vi "AeroQuadConfigurator.vi"() -> ()   [LabVIEW 2010]
uses:
  <vilib>/Utility/config.llb/Config Data RefNum.ctl
  <vilib>/Utility/miscctls.llb/LVRowAndColumnTypeDef.ctl
  <vilib>/Utility/miscctls.llb/LVRowAndColumnUnsignedTypeDef.ctl
  <vilib>/Utility/config.llb/Read Key (Double).vi
  <vilib>/Utility/config.llb/Read Key (String).vi
  <vilib>/Utility/config.llb/Read Key (I32).vi
  <vilib>/Utility/config.llb/Write Key (I32).vi
  <vilib>/Utility/config.llb/Write Key (String).vi
  <vilib>/Platform/browser.llb/Open URL in Default Browser (string).vi
  <vilib>/Instr/_visa.llb/VISA Configure Serial Port (Instr).vi
  <vilib>/Utility/config.llb/NI_LVConfig.lvlib
panel:
  out "LargeStatus":string
  in  "Load SubPanel":i32(ring) caption="Information Display" items=["Initial Setup", "3-D View", "Vehicle Status", "Mission Planner", "Motor Commands", "Serial Monitor", "Vehicle Attitude", "Sensor Data", "Transmitter Data"]
  in  "Parameter Type":i32(ring) caption="Configuration" items=["Rate Mode", "Attitude Mode", "Yaw Configuration", "Altitude Hold", "GPS Position Hold", "Miscellaneous Configuration", "Transmitter Smoothing", "Battery Monitor", "Camera Stabilization"]
  in  "Parameter Check":string[][](table)
  in  "Upload":bool
  out "Sensors":string[][](table)
  out "Status":string="AeroQuad Configurator"
  in  "*Com Port":refnum<visa-resource-name> caption="Com Port"
  in  "*Baud Rate":string(combo)="115200" caption="Baud Rate"
  in  "*BootDelay":dbl=3.0 caption="Boot Delay (s)"
  in  "*Timeout (sec)":dbl=3.0 caption="Timeout (s)"
  in  "Open Port":bool
  in  "Disconnect":bool
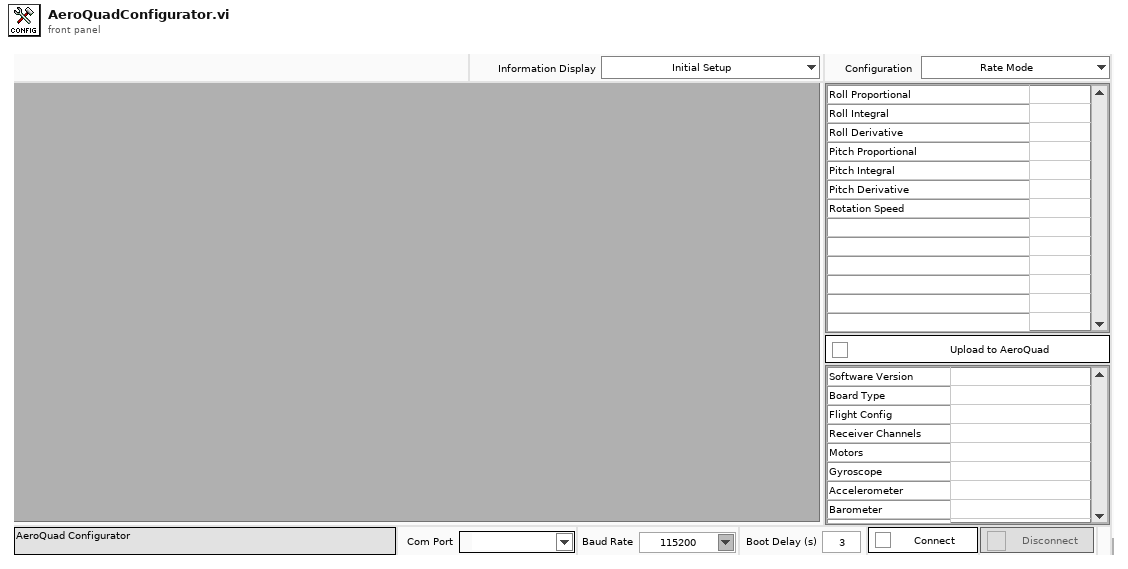
[diagram p1: front panel]
types:
  T1 = typedef "NI_LVConfig.lvlib/Config Data RefNum.ctl" = refnum<k1>
  T2 = cluster{"Error":errorcluster, "Data":dbl[], "COM Port":refnum<visa-resource-name>, "Data Type":enum16{"Serial", "Binary"}, "Connected":bool, "Parameters":string[][][], "WorkingPath":path, "ConfigRef":T1, "SubPanelName":string[], "ParameterName":string[], "Plots":string[][][], "SubPanelQueue":refnum<queue>, "SubPanel":refnum<vi>, "Debug":bool, "SubPanelType":string[], "Version":string, "StopTelem":string, "Config":string[][], "oldTelem":string, "previousValid":string, "oldCmd":string, "StartDelay":dbl, "ParamDesc":string[][], "IniPath":path, "SW":string, "ConnType":string, "ModemQueue":refnum<queue>, "Stale":i32, "Compatibility":dbl, "Logger":bool, "DebugLogger":refnum<queue>}
  T3 = enum8{"Enabled", "Disabled", "Disabled and Grayed Out"}
  T4 = cluster{"Section":string, "Key":string, "Value":string}
  T5 = enum32{"Invalid", "Standard", "Closed", "Hidden", "Minimized", "Maximized"}
  T6 = typedef "LVRowAndColumnTypeDef.ctl" = cluster{"Row":i32, "Column":i32}
  T7 = typedef "LVRowAndColumnUnsignedTypeDef.ctl" = cluster{"Row":u32, "Column":u32}
  T8 = enum32{"invalid app kind", "Development System", "Run Time System", "Student Edition", "Embedded LabVIEW", "Evaluation", "Custom"}
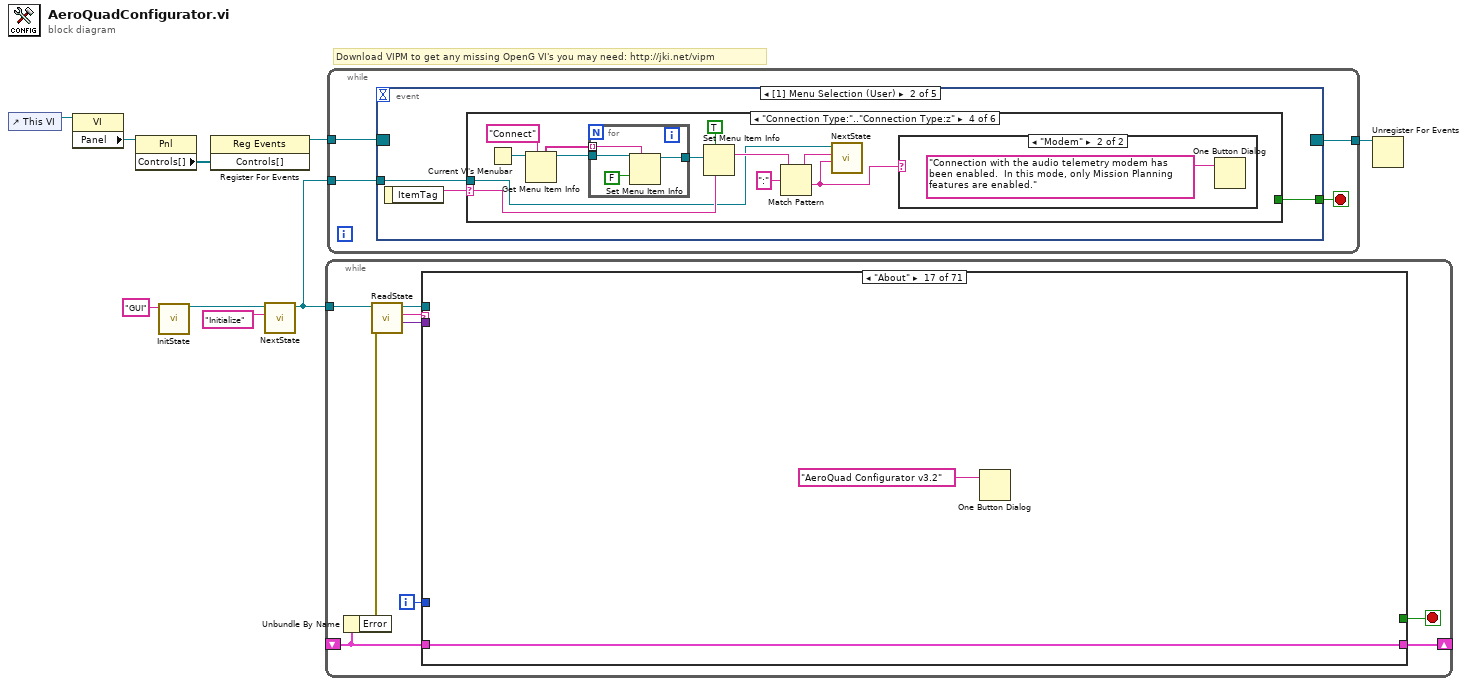
[diagram p0: block diagram]
diagram:
  # "Download VIPM to get any missing OpenG VI's you may need: http://jki.net/vipm"
  n1 = control-ref of="This VI"() -> (w9:refnum<vi>)
  n2 = property class="VI"(reference=w9) -> ("Panel"=w8:refnum<vi>)  [unwired: 1 in, 2 out]
  n3 = property class="Pnl"(reference=w8) -> ("Controls[]"=w7:refnum<vi>[])  [unwired: 1 in, 2 out]
  n4 = call "InitState.vi"("Name"="GUI") -> ("Queue Out"=w2:refnum<queue>)  [unwired: 8 in, 1 out]
  n5 = register-events(w7) -> (reference out=w6:refnum<event-registration>)  [unwired: 2 in, 1 out]
  n6 = call "NextState.vi"("State"="Initialize", "Queue In"=w2) -> ("Queue Out"=w3:refnum<queue>)  [unwired: 8 in, 1 out]
  n7 = while {
    tunnel: w3 -> [w13]
    shift-right: [w18] -> _
    shift-left: _ -> [w15]
    i -> [w16]
    stop <- w17 stop-if-true
    n8 = Unbundle By Name(w15) -> ("Error"=w14:errorcluster)
    n9 = call "ReadState.vi"("Error In"=w14, "Queue In"=w13) -> ("Data"=w10:variant, "State"=w11:string, "Queue Out"=w12:refnum<queue>)  [unwired: 6 in, 1 out]
    n10 = case shown="\"About\"" w11 {
      tunnel: w10 -> [_ _ _ w51 _ _ _ _ _ _ _ _ _ w251 w266 _ _ _ w323 w329 _ _ _ _ _ _ _ _ _ w492 w496 _ _ _ w667 _ _ _ w775 _ w785 _ _ w871 _ _ _ _ _ w1079 _ w1165 _ _ _ _ _ _ _ _ w1351 _ _ _ w1494 w1509 _ _ w1626 w1654 w1722]
      selector: w11 -> [_ w22 _ _ _ _ _ _ _ _ _ _ _ _ w256 _ _ _ _ _ _ _ _ _ _ _ _ _ _ _ _ _ _ _ w663 _ _ _ _ _ _ _ _ _ _ _ _ _ _ w1078 _ _ _ _ _ _ _ _ _ _ _ _ _ _ _ _ _ _ w1625 w1653 _]
      tunnel: [w19 w23 w36 w52 w56 w75 w111 w171 w187 w191 w193 w204 w240 w253 w267 w285 w317 w320 w324 w330 w332 w343 w346 w381 w436 w437 w470 w485 w487 w491 w497 w516 w544 w622 w668 w691 w726 w757 w772 w781 w787 w806 w818 w868 w903 w917 w949 w968 w1055 w1092 w1150 w1163 w1178 w1179 w1185 w1213 w1237 w1262 w1289 w1318 w1353 w1421 w1427 w1429 w1497 w1557 w1563 w1600 w1623 w1651 w1728] -> w18
      tunnel: [_ _ _ _ _ _ _ _ _ _ _ _ _ _ _ _ _ _ _ _ _ TRUE _ _ _ _ _ _ _ _ _ _ _ _ _ _ _ _ _ _ _ _ _ _ _ _ _ _ _ _ _ _ _ _ _ _ _ _ _ _ _ _ _ _ _ _ _ _ _ _ _] -> w17
      tunnel: w15 -> [w19 w23 _ w52 w56 w75 w112 w172 w188 w191 w193 w205 w241 w254 w267 w286 w317 w320 w324 w330 w332 w343 w346 w382 w436 w438 w470 w485 w487 w491 w497 w503 w545 w596 w669 w692 w727 w758 w772 w781 w788 w807 w819 w865 w903 w917 w949 w969 w1056 w1093 w1150 w1163 w1178 w1179 w1186 w1214 w1238 w1263 w1290 w1319 w1354 w1421 w1427 w1430 w1497 w1557 w1563 w1600 w1624 w1651 w1728]
      tunnel: w16 -> [_ _ _ _ _ _ _ _ _ _ _ _ _ _ _ w287 _ _ _ _ _ _ _ _ _ _ _ _ _ _ _ _ _ _ _ _ _ _ _ _ _ _ _ _ _ _ _ _ _ _ _ _ _ _ _ _ _ _ _ _ _ _ _ _ _ _ _ _ _ _ _]
      tunnel: w12 -> [_ _ w47 _ _ _ _ _ _ _ _ w198 w231 _ w260 w283 _ w319 _ _ _ w344 _ w355 _ _ _ _ _ _ w493 w508 w546 w621 w664 _ w725 w754 _ _ w789 w815 w825 w866 _ _ _ _ _ w1074 w1107 _ w1167 _ w1183 w1211 _ _ w1284 w1315 w1348 w1415 _ w1431 w1492 w1522 _ _ _ w1648 w1727]
      frame "--- System ---" {
      }
      frame Default {
        n11 = Format Into String(format string="Invalid state:\n%s", w22) -> (resulting string=w20:string)  [unwired: 2 in, 1 out]
        n12 = One Button Dialog(message=w20) -> ()  [unwired: 1 in, 1 out]
      }
      frame "Initialize" {
        w27 = "Launch" ("name (unnamed)")
        w28 = T3."Enabled" ("Disabled")
        # "Used for splash screen"
        n13 = call "NextState.vi"("Data"="Initializing Configurator", "State"="Status", "Queue In"=w47) -> ("Queue Out"=w30:refnum<queue>)  [unwired: 7 in, 1 out]
        n14 = call "NextStates.vi"("States"=string[] ["Lock Controls", "Load Config", "Load Parameters", "Load SubPanels", "Load Front Panel"], "Queue In"=w30) -> ("Queue Out"=w29:refnum<queue>)  [unwired: 8 in, 1 out]
        n15 = Current VI's Path() -> (path=w39:path)
        n16 = property class="App"() -> ("App.Kind"=w41:T8)  [unwired: 2 in, 2 out]
        n17 = call "NextState.vi"("Data"="Configurator Ready - Waiting to Connect", "State"="Status", "Queue In"=w29) -> ("Queue Out"=w35:refnum<queue>)  [unwired: 7 in, 1 out]
        n18 = Strip Path(path=w39) -> (stripped path=w40:path)  [unwired: 1 out]
        n19 = local write "Sensors"(string[][] [] ("Sensors")) -> ()
        n20 = case shown="\"Run Time System\", Default" w41 {
          tunnel: w40 -> [w48 w50]
          tunnel: [w48 w49] -> w38
          frame "Development System" {
          }
          frame "Run Time System", Default {
            n21 = Strip Path(path=w50) -> (stripped path=w49:path)  [unwired: 1 out]
          }
        }
        n22 = Obtain Notifier(name (unnamed)=w27, notification data type=w27, create if not found? (T)=FALSE) -> (notifier out=w25:refnum<notifier>)  [unwired: 1 in, 2 out]
        n23 = Send Notification(notification="Done", notifier=w25) -> ()  [unwired: 1 in, 2 out]
        n24 = call "NextState.vi"("State"="Unlock Comm Controls", "Queue In"=w35) -> ("Queue Out"=w33:refnum<queue>)  [unwired: 8 in, 1 out]
        n25 = property on="Parameter Type" class="Ring (strict)"("DisabledEnum"=w28) -> ()  [unwired: 2 in, 2 out]
        n26 = property on="Load SubPanel" class="Ring (strict)"("DisabledEnum"=w28) -> ()  [unwired: 2 in, 2 out]
        n27 = Bundle By Name(cluster=T2 {"Error"={"status"=FALSE, "code"=0, "source"=""}, "Data"=[0.0, 0.0, 0.0, 0.0, 0.0, 0.0, 0.0, 0.0, 0.0, 0.0, 0.0, 0.0, 0.0, 0.0, 0.0, 0.0, 0.0, 0.0, 0.0, 0.0, 0.0, 0.0, 0.0, 0.0, 0.0, 0.0, 0.0, 0.0, 0.0, 0.0, 0.0, 0.0], "COM Port"="COM2", "Data Type"=enum."Serial", "Connected"=FALSE, "Parameters"=[], "WorkingPath"=path "", "ConfigRef"=refnum, "SubPanelName"=[], "ParameterName"=[], "Plots"=[], "SubPanelQueue"=refnum, "SubPanel"=refnum, "Debug"=FALSE, "SubPanelType"=[], "Version"="", "StopTelem"="", "Config"=[], "oldTelem"="", "previousValid"="", "oldCmd"="", "StartDelay"=0.0, "ParamDesc"=[], "IniPath"=path "", "SW"="", "ConnType"="Check Connection", "ModemQueue"=refnum, "Stale"=0, "Compatibility"=3.1, "Logger"=FALSE, "DebugLogger"=refnum}, "WorkingPath"=w38) -> (w36:T2)
        n28 = property on="Upload" class="Bool"("DisabledEnum"=w28) -> ()  [unwired: 2 in, 2 out]
        n29 = call "NextState.vi"("State"="Unlock User Controls", "Queue In"=w33) -> ()  [unwired: 8 in, 2 out]
      }
      frame "Status" {
        n30 = Variant To Data(Variant=w51, type="") -> (data=→"Status":string)  [unwired: 1 in, 1 out]
      }
      frame "Lock Controls" {
        n31 = control-ref of="This VI"() -> (w63:refnum<vi>)
        n32 = property class="VI"(reference=w63) -> ("Panel"=w64:refnum<vi>)  [unwired: 1 in, 2 out]
        n33 = property class="Pnl"(reference=w64) -> ("Controls[]"=w59:refnum<vi>[])  [unwired: 1 in, 2 out]
        n34 = for {
          tunnel: w59 -> [w67] mode=indexing
          tunnel: [w68] -> w62 mode=indexing
          tunnel: T3."Disabled and Grayed Out" ("Disabled") -> [w65]
          n35 = property class="Ctl"(reference=w67) -> ("ClassID"=w66:u32)  [unwired: 1 in, 2 out]
          n36 = case shown="8" w66 {
            tunnel: [w69 w73] -> w68
            tunnel: w67 -> [w70 w72]
            tunnel: w65 -> [_ w71]
            frame Default {
              n37 = property class="Ctl"(reference=w70) -> ("Label.Text"=w69:string)  [unwired: 1 in, 2 out]
            }
            frame 8 {
              n38 = property class="Ctl"(reference=w72, "DisabledEnum"=w71) -> ("Label.Text"=w73:string)  [unwired: 1 in, 2 out]
            }
          }
        }
        n39 = Search 1D Array(1D array=w62, element="Open Port") -> (index of element=w60:i32)  [unwired: 1 in]
        n40 = Index Array(array=w59, index=w60) -> (element=w58:refnum<vi>)
        n41 = property class="Ctl"(reference=w58, "DisabledEnum"=T3."Enabled" ("Disabled")) -> ()  [unwired: 1 in, 2 out]
      }
      frame "Unlock Controls" {
        n42 = control-ref of="This VI"() -> (w82:refnum<vi>)
        n43 = property class="VI"(reference=w82) -> ("Panel"=w83:refnum<vi>)  [unwired: 1 in, 2 out]
        n44 = property class="Pnl"(reference=w83) -> ("Controls[]"=w78:refnum<vi>[])  [unwired: 1 in, 2 out]
        n45 = for {
          tunnel: w78 -> [w86] mode=indexing
          tunnel: [w87] -> w81 mode=indexing
          tunnel: T3."Enabled" ("Disabled") -> [w84]
          n46 = property class="Ctl"(reference=w86) -> ("ClassID"=w85:u32)  [unwired: 1 in, 2 out]
          n47 = case shown="8" w85 {
            tunnel: [w88 w92] -> w87
            tunnel: w86 -> [w89 w91]
            tunnel: w84 -> [_ w90]
            frame Default {
              n48 = property class="Ctl"(reference=w89) -> ("Label.Text"=w88:string)  [unwired: 1 in, 2 out]
            }
            frame 8 {
              n49 = property class="Ctl"(reference=w91, "DisabledEnum"=w90) -> ("Label.Text"=w92:string)  [unwired: 1 in, 2 out]
            }
          }
        }
        n50 = Search 1D Array(1D array=w81, element="Open Port") -> (index of element=w79:i32)  [unwired: 1 in]
        n51 = Index Array(array=w78, index=w79) -> (element=w77:refnum<vi>)
        n52 = property class="Ctl"(reference=w77, "DisabledEnum"=T3."Disabled and Grayed Out" ("Disabled")) -> ()  [unwired: 1 in, 2 out]
      }
      frame "Load Config" {
        w98 = string[] []
        # "Get type of data found in configuration file:\n1) Configuration Parameters\n2) Custom Plots"
        n53 = Unbundle By Name(w112) -> ("WorkingPath"=w110:path)
        n54 = property class="App"() -> ("App.Kind"=w100:T8)  [unwired: 2 in, 2 out]
        n55 = case shown="\"Run Time System\"" w100 {
          tunnel: [w116 "AeroQuadConfigurator.ini" ("name or relative path")] -> w101
          frame "Run Time System" {
            n56 = property class="App"() -> ("OS.Name"=w122:string)  [unwired: 2 in, 2 out]
            n57 = Match Pattern(string=w122, regular expression="Mac") -> (offset past match=w120:i32)  [unwired: 1 in, 3 out]
            n58 = Greater Or Equal To 0?(x=w120) -> (x >= 0?=w119:bool)
            n59 = Select(t="AeroQuad Configurator preferences" ("name or relative path"), s=w119, f="AeroQuadConfigurator.ini" ("name or relative path")) -> (s? t:f=w116:string)
          }
          frame "Development System", Default {
          }
        }
        n60 = Build Path(base path=w110, name or relative path=w101) -> (appended path=w93:path)
        n61 = call <vilib>:"Open Config Data.vi"("create file if necessary (T)"=FALSE, "configuration file path"=w93) -> ("error out"=w113:errorcluster, "refnum"=w114:T1)  [unwired: 7 in, 1 out]
        n62 = call <vilib>:"Get Section Names.vi"("error in (no error)"=w113, "refnum"=w114) -> ("error out"=w107:errorcluster, "section names"=w108:string[], "refnum out"=w109:T1)  [unwired: 7 in]
        n63 = for {
          tunnel: w109 -> [w138]
          tunnel: w108 -> [w127] mode=indexing
          shift-right: [w134] -> w104
          shift-left: w107 -> [w136]
          tunnel: [w132] -> w94
          shift-right: [w131] -> w106
          shift-left: w98 -> [w130]
          shift-right: [w128] -> w105
          shift-left: w98 -> [w129]
          shift-right: [w124] -> w99
          shift-left: w98 -> [w125]
          n64 = call-poly <vilib>:"Read Key.vi"("section"=w127, "error in (no error)"=w136, "key"="Type", "refnum"=w138) -> ("error out"=w135:errorcluster, "value"=w126:string, "refnum out"=w133:T1)  [unwired: 4 in, 1 out]
          n65 = case shown="\"Parameters\"" w126 {
            selector: w126 -> [_ w147 w156 _]
            tunnel: [w142 w153 w162 w168] -> w134
            tunnel: w135 -> [w142 w153 w162 w168]
            tunnel: [w143 w154 w163 w167] -> w132
            tunnel: w133 -> [w143 w154 w163 w167]
            tunnel: [w145 w150 w159 w166] -> w131
            tunnel: w130 -> [w144 w150 w159 w166]
            tunnel: [w141 w151 w160 w165] -> w128
            tunnel: w129 -> [w141 w152 w161 w165]
            tunnel: w127 -> [w140 w149 w158 _]
            tunnel: w125 -> [w139 w148 w157 w164]
            tunnel: [w139 w146 w155 w164] -> w124
            frame "Parameters" {
              n66 = Build Array (concatenate)(w144, w140) -> (w145:string[])
            }
            frame "Binary Plot", "Plot" {
              n67 = Build Array (concatenate)(w152, w149) -> (w151:string[])
              n68 = Build Array (concatenate)(w148, w147) -> (w146:string[])
            }
            frame "Module" {
              n69 = Build Array (concatenate)(w161, w158) -> (w160:string[])
              n70 = Build Array (concatenate)(w157, w156) -> (w155:string[])
            }
            frame Default {
            }
          }
        }
        n71 = Path To String(path=w93) -> (string=w102:string)
        n72 = Bundle By Name(cluster=w104, "source"=w102) -> (w103:errorcluster)
        n73 = call-poly <vilib>:"Read Key.vi"("section"="Configuration", "key"="StartUpDelay", "refnum"=w94) -> ("value"=w95:dbl)  [unwired: 5 in, 3 out]
        n74 = Bundle By Name(cluster=w112, "StartDelay"=w95, "SubPanelType"=w99, "SubPanelName"=w105, "ParameterName"=w106, "Error"=w103, "ConfigRef"=w94, "IniPath"=w93) -> (w111:T2)
      }
      frame "Load Front Panel" {
        w169 = "Configuration" ("section")
        n75 = Unbundle By Name(w172) -> ("ConfigRef"=w178:T1)
        n76 = call-poly <vilib>:"Read Key.vi"("section"=w169, "key"="SubPanel", "refnum"=w178) -> ("value"=w176:i32, "refnum out"=w174:T1)  [unwired: 5 in, 2 out]
        n77 = local write "Load SubPanel"(w176) -> ()
        n78 = call-poly <vilib>:"Read Key.vi"("section"=w169, "key"="Parameter", "refnum"=w174) -> ("error out"=w170:errorcluster, "value"=w173:i32)  [unwired: 5 in, 2 out]
        n79 = local write "Parameter Type"(w173) -> ()
        n80 = Bundle By Name(cluster=w172, "Error"=w170) -> (w171:T2)
      }
      frame "Save Front Panel" {
        w182 = "Configuration" ("section")
        n81 = Unbundle By Name(w188) -> ("ConfigRef"=w189:T1)
        n82 = local read "Load SubPanel"() -> (w185:i32)
        n83 = call-poly <vilib>:"Write Key.vi"("section"=w182, "value"=w185, "key"="SubPanel", "refnum"=w189) -> ("error out"=w180:errorcluster, "refnum out"=w183:T1)  [unwired: 5 in, 1 out]
        n84 = local read "Parameter Type"() -> (w181:i32)
        n85 = call-poly <vilib>:"Write Key.vi"("section"=w182, "error in (no error)"=w180, "value"=w181, "key"="Parameter", "refnum"=w183) -> ("error out"=w179:errorcluster)  [unwired: 4 in, 2 out]
        n86 = Bundle By Name(cluster=w188, "Error"=w179) -> (w187:T2)
      }
      frame "Lock User Controls" {
        w190 = T3."Disabled and Grayed Out" ("Disabled")
        n87 = property on="Parameter Type" class="Ring (strict)"("DisabledEnum"=w190) -> ()  [unwired: 2 in, 2 out]
        n88 = property on="Load SubPanel" class="Ring (strict)"("DisabledEnum"=w190) -> ()  [unwired: 2 in, 2 out]
        n89 = property on="Upload" class="Bool"("DisabledEnum"=w190) -> ()  [unwired: 2 in, 2 out]
      }
      frame "Unlock User Controls" {
        w192 = T3."Enabled" ("Disabled")
        n90 = property on="Parameter Type" class="Ring (strict)"("DisabledEnum"=w192) -> ()  [unwired: 2 in, 2 out]
        n91 = property on="Load SubPanel" class="Ring (strict)"("DisabledEnum"=w192) -> ()  [unwired: 2 in, 2 out]
        n92 = property on="Upload" class="Bool"("DisabledEnum"=w192) -> ()  [unwired: 2 in, 2 out]
      }
      frame "Load Parameters" {
        # "Index for ParameterName\nand Parameters are the same."
        n93 = Unbundle By Name(w205) -> ("ParameterName"=w199:string[], "ConfigRef"=w202:T1)
        n94 = call "NextState.vi"("State"="Update Comm Controls", "Queue In"=w198) -> ("Queue Out"=w197:refnum<queue>)  [unwired: 8 in, 1 out]
        n95 = property on="Parameter Type" class="Ring (strict)"("Strings []"=w199) -> ()  [unwired: 2 in, 2 out]
        n96 = for {
          shift-right: [w210] -> w195
          shift-left: errorcluster {"status"=FALSE, "code"=0, "source"=""} ("error out") -> [w216]
          tunnel: w202 -> [w215]
          tunnel: w199 -> [w212] mode=indexing
          tunnel: [w211] -> w200 mode=indexing
          tunnel: [w206] -> w194 mode=indexing
          n97 = call <vilib>:"Get Key Names.vi"("section"=w212, "error in (no error)"=w216, "refnum"=w215) -> ("error out"=w214:errorcluster, "key names"=w209:string[], "refnum out"=w213:T1)  [unwired: 5 in, 1 out]
          n98 = Split 1D Array(array=w209, index=1) -> (second subarray=w207:string[])  [unwired: 1 out]
          n99 = for {
            shift-right: [w222] -> w210
            shift-left: w214 -> [w226]
            tunnel: w213 -> [w225]
            tunnel: w207 -> [w223] mode=indexing
            tunnel: w212 -> [w224]
            tunnel: [w221] -> w211 mode=indexing
            tunnel: [w217] -> w206 mode=indexing
            n100 = call-poly <vilib>:"Read Key.vi"("section"=w224, "error in (no error)"=w226, "key"=w223, "refnum"=w225) -> ("error out"=w222:errorcluster, "value"=w220:string)  [unwired: 4 in, 2 out]
            n101 = Match Pattern(string=w220, regular expression=",") -> (before substring=w218:string, after substring=w217:string)  [unwired: 1 in, 2 out]
            n102 = Build Array(w223, w218) -> (w221:string[])
          }
        }
        n103 = call "NextState.vi"("State"="Parameter Type", "Queue In"=w197) -> ()  [unwired: 8 in, 2 out]
        n104 = Bundle By Name(cluster=w205, "Parameters"=w200, "ParamDesc"=w194, "Error"=w195) -> (w204:T2)
      }
      frame "Load SubPanels" {
        w228 = 32  # Buffers
        w229 = "Modem Telemetry" ("name (unnamed)")
        # "Convenient place to initialize\nmodem queue."
        # "Load SubPanel names, add custom plots at end."
        n105 = call "NextState.vi"("State"="Load SubPanel", "Queue In"=w231) -> ()  [unwired: 8 in, 2 out]
        n106 = Unbundle By Name(w241) -> ("SubPanelName"=w230:string[], "ConfigRef"=w234:T1)
        n107 = for {
          tunnel: w234 -> [w245]
          tunnel: [w244] -> w233 mode=indexing
          tunnel: w230 -> [w242] mode=indexing
          tunnel: [w243] -> w232 mode=indexing
          n108 = call "GetSectionData.vi"("SectionName"=w242, "ConfigRef"=w245) -> ("error out"=w244:errorcluster, "Data"=w243:string[][])  [unwired: 7 in, 1 out]
        }
        n109 = property on="Load SubPanel" class="Ring (strict)"("Strings []"=w230) -> ()  [unwired: 2 in, 2 out]
        n110 = Merge Errors(w233) -> (w239:errorcluster)
        n111 = Obtain Queue(max queue size (-1, unlimited)=w228, name (unnamed)=w229, element data type=w229) -> (queue out=w227:refnum<queue>)  [unwired: 2 in, 2 out]
        n112 = Obtain Queue(name (unnamed)="SubPanel", element data type=cluster{"State":string, "Data":variant} {"State"="", "Data"=variant}) -> (queue out=w235:refnum<queue>)  [unwired: 3 in, 2 out]
        n113 = Bundle By Name(cluster=w241, "ModemQueue"=w227, "Plots"=w232, "Error"=w239, "SubPanelQueue"=w235) -> (w240:T2)
      }
      frame "Save Configuration" {
        n114 = Variant To Data(Variant=w251, type=T4 {"Section"="", "Key"="", "Value"=""}) -> (data=w249:T4)  [unwired: 1 in, 1 out]
        n115 = Unbundle By Name(w249) -> ("Section"=w248:string, "Key"=w247:string, "Value"=w246:string)
        n116 = Unbundle By Name(w254) -> ("ConfigRef"=w255:T1)
        n117 = call-poly <vilib>:"Write Key.vi"("section"=w248, "value"=w246, "key"=w247, "refnum"=w255) -> ("error out"=w252:errorcluster)  [unwired: 5 in, 2 out]
        n118 = Bundle By Name(cluster=w254, "Error"=w252) -> (w253:T2)
      }
      frame "Menu Link" {
        w265 = "199.193.247.52"  # www.AeroQuad.com
        n119 = Variant To Data(Variant=w266, type=w256) -> (data=w257:string)  [unwired: 1 in, 1 out]
        n120 = case shown="\"Bug Reporting\"" w257 {
          tunnel: ["https://aeroquad.atlassian.net" ("URL") "http://aeroquad.com/showwiki.php?title=AeroQuad+3+x+Configurator+Manual" ("URL") "http://aeroquad.com/showwiki.php" ("URL") "http://aeroquad.com/forum.php" ("URL")] -> w258
          frame "Bug Reporting" {
          }
          frame "User Manual" {
          }
          frame "Documentation" {
          }
          frame "Forum", Default {
          }
        }
        n121 = TCP Open Connection(address=w265, remote port or service name=u16 80, timeout ms (60000)=3000) -> (connection ID=w261:refnum<k5>, error out=w262:errorcluster)  [unwired: 2 in]
        n122 = TCP Close Connection(connection ID=w261, error in (no error)=w262) -> (error out=w259:errorcluster)  [unwired: 1 in, 1 out]
        n123 = case shown="Error" w259 {
          tunnel: w260 -> [_ w271]
          tunnel: w258 -> [w268 _]
          tunnel: w257 -> [_ w270]
          tunnel: w256 -> [_ w269]
          frame No Error {
            n124 = call-poly <vilib>:"Open URL in Default Browser.vi"("URL"=w268) -> ()  [unwired: 5 in, 2 out]
          }
          frame Error {
            n125 = Two Button Dialog(message="This feature requires a network connection.", 2:"Retry" ("T button name (\"OK\")")) -> (T button?=w272:bool)  [unwired: 1 in]
            n126 = case shown="False" w272 {
              tunnel: w271 -> [_ w277]
              tunnel: w269 -> [_ w276]
              tunnel: w270 -> [_ w275]
              frame False {
              }
              frame True {
                n127 = call "NextState.vi"("Data"=w275, "State"=w276, "Queue In"=w277) -> ()  [unwired: 7 in, 2 out]
              }
            }
          }
        }
      }
      frame "Error" {
        n128 = Flush Queue(queue=w283) -> (queue out=w284:refnum<queue>)  [unwired: 1 in, 2 out]
        n129 = case shown="Default" w287 {
          tunnel: w286 -> [w289 w293]
          tunnel: [w288 w295] -> w285
          tunnel: w284 -> [_ w294]
          frame 0 {
            n130 = in-place {
              n131 = in-place-cluster #1(w289) -> ("Error"=w291:errorcluster)
              n132 = call <vilib>:"Clear Errors.vi"("error in (no error)"=w291) -> ("error out"=w290:errorcluster)  [unwired: 6 in]
              n133 = in-place-cluster #1("Error"=w290) -> (w288:T2)
            }
          }
          frame Default {
            n134 = Unbundle By Name(w293) -> ("Error.code"=w292:i32)
            n135 = case shown="7, 1003" w292 {
              tunnel: w293 -> [w302 w309]
              tunnel: [w301 w308] -> w295
              tunnel: w294 -> [w298 w307]
              frame 7, 1003 {
                n136 = Unbundle By Name(w302) -> ("Error"=w296:errorcluster)
                n137 = call "NextState.vi"("State"="Load SubPanel", "Queue In"=w298) -> ()  [unwired: 8 in, 2 out]
                n138 = call <vilib>:"Clear Errors.vi"("error in (no error)"=w296) -> ("error out"=w300:errorcluster)  [unwired: 6 in]
                n139 = Bundle By Name(cluster=w302, "Error"=w300) -> (w301:T2)
                n140 = local write "Load SubPanel"(0) -> ()
                n141 = One Button Dialog(message="This feature is currently not supported in this version of the Configurator") -> ()  [unwired: 1 in, 1 out]
              }
              frame Default {
                n142 = in-place {
                  in-place-border: [w313] -> w304
                  n143 = in-place-cluster #2(w309) -> ("Connected"=w313:bool, "Error"=w315:errorcluster)
                  n144 = call "ErrorDialog.vi"("error in"=w315) -> ("error out"=w314:errorcluster)  [unwired: 10 in]
                  n145 = call <vilib>:"Clear Errors.vi"("error in (no error)"=w314) -> ("error out"=w316:errorcluster)  [unwired: 6 in]
                  n146 = in-place-cluster #2("Connected"=FALSE, "Error"=w316) -> (w308:T2)
                }
                n147 = call "NextState.vi"("State"="Disconnect", "Queue In"=w307) -> ("Queue Out"=w305:refnum<queue>)  [unwired: 8 in, 1 out]
                n148 = case shown="True" w304 {
                  tunnel: w305 -> [_ w311]
                  frame False {
                  }
                  frame True {
                    n149 = call "NextState.vi"("State"="Reconnect", "Queue In"=w311) -> ()  [unwired: 8 in, 2 out]
                  }
                }
              }
            }
          }
        }
        n150 = local write "Status"("Error detected!" ("Status")) -> ()
      }
      frame "About" {
        n151 = One Button Dialog(message="AeroQuad Configurator v3.2") -> ()  [unwired: 1 in, 1 out]
      }
      frame "Clear Queue" {
        n152 = Flush Queue(queue=w319) -> ()  [unwired: 1 in, 3 out]
      }
      frame "Delay" {
        n153 = Variant To Data(Variant=w323, type=u32 0 ("milliseconds to wait")) -> (data=w321:u32)  [unwired: 1 in, 1 out]
        n154 = Wait (ms)(milliseconds to wait=w321) -> ()  [unwired: 1 out]
      }
      frame "Delay String" {
        n155 = Variant To Data(Variant=w329, type="") -> (data=w327:string)  [unwired: 1 in, 1 out]
        n156 = Decimal String To Number(string=w327) -> (number=w326:i32)  [unwired: 2 in, 1 out]
        n157 = To Unsigned Long Integer(number=w326) -> (unsigned 32bit integer=w325:u32)
        n158 = Wait (ms)(milliseconds to wait=w325) -> ()  [unwired: 1 out]
      }
      frame "Delay SubPanel" {
        n159 = Wait (ms)(milliseconds to wait=u32 250) -> ()  [unwired: 1 out]
      }
      frame "Exit" {
        n160 = Unbundle By Name(w343) -> ("ModemQueue"=w333:refnum<queue>, "Debug"=w337:bool, "SubPanel"=w339:refnum<vi>, "SubPanelQueue"=w340:refnum<queue>, "ConfigRef"=w342:T1, "COM Port"=w336:refnum<visa-resource-name>, "StopTelem"=w334:string)
        n161 = Release Queue(queue=w344) -> ()  [unwired: 2 in, 3 out]
        n162 = Release Queue(queue=w333) -> ()  [unwired: 2 in, 3 out]
        n163 = VISA Write(VISA resource name=w336, write buffer=w334) -> (VISA resource name out=w335:refnum<visa-resource-name>)  [unwired: 1 in, 2 out]
        n164 = VISA Close(VISA resource name=w335) -> ()  [unwired: 1 in, 1 out]
        n165 = call <vilib>:"Close Config Data.vi"("write file if changed (T)"=TRUE, "refnum"=w342) -> ()  [unwired: 8 in, 2 out]
        n166 = Release Queue(queue=w340) -> ()  [unwired: 2 in, 3 out]
        n167 = invoke class="VI" method="Abort VI"(reference=w339) -> (reference out=w338:refnum<vi>)  [unwired: 2 in, 2 out]
        n168 = Close Reference(reference=w338) -> ()  [unwired: 1 in, 1 out]
        n169 = case shown="False" w337 {
          frame False {
            n170 = invoke class="VI" method="FP.Close"() -> ()  [unwired: 3 in, 3 out]
          }
          frame True {
          }
        }
      }
      frame "--- GUI ---" {
      }
      frame "Load SubPanel" {
        w347 = T3."Enabled" ("Disabled")
        # "Close previous panel."
        n171 = Unbundle By Name(w382) -> ("Config"=w348:string[][], "SubPanelType"=w353:string[], "ConfigRef"=w376:T1, "Plots"=w373:string[][][], "SubPanelName"=w351:string[], "WorkingPath"=w362:path, "SubPanelQueue"=w367:refnum<queue>, "COM Port"=w358:refnum<visa-resource-name>, "SubPanel"=w359:refnum<vi>)
        n172 = flat-sequence {
          tunnel: w359 -> [w387]
          tunnel: w358 -> [w386]
          tunnel: w355 -> [w384]
          tunnel: [w383] -> w357
          frame #0 {
            n173 = invoke class="VI" method="Abort VI"(reference=w387) -> (reference out=w388:refnum<vi>)  [unwired: 2 in, 2 out]
            n174 = Close Reference(reference=w388) -> ()  [unwired: 1 in, 1 out]
            n175 = VISA Write(VISA resource name=w386, write buffer="X") -> ()  [unwired: 1 in, 3 out]
            n176 = Flush Queue(queue=w384) -> (error out=w383:errorcluster)  [unwired: 1 in, 2 out]
          }
        }
        n177 = property on="Load SubPanel" class="Ring (strict)"() -> ("Strings []"=w377:string[])  [unwired: 2 in, 2 out]
        n178 = Index Array(array=w377, index="Load SubPanel") -> (element=w350:string)
        n179 = Search 1D Array(1D array=w351, element=w350) -> (index of element=w349:i32)  [unwired: 1 in]
        n180 = Index Array(array=w353, index=w349) -> (element=w354:string)
        n181 = property class="App"() -> ("App.Kind"=w365:T8)  [unwired: 2 in, 2 out]
        n182 = Flush Queue(queue=w367, error in (no error)=w357) -> (error out=w366:errorcluster)  [unwired: 2 out]
        n183 = case shown="\"Module\"" w354 {
          tunnel: w350 -> [_ w397 _ _]
          tunnel: w376 -> [_ w403 _ _]
          tunnel: w373 -> [_ _ w417 w430]
          tunnel: [_ w398 w416 w429] -> w372
          tunnel: [_ w399 _ _] -> w369
          tunnel: w365 -> [_ w396 w414 w427]
          tunnel: w362 -> [_ _ _ _]
          tunnel: [_ w395 w415 w428] -> w361
          tunnel: w349 -> [_ _ w413 w426]
          tunnel: w348 -> [_ w390 w412 w423]
          frame Default {
            n184 = One Button Dialog(message="Unknown module type. \nVerify INI file is correctly configured.") -> ()  [unwired: 1 in, 1 out]
          }
          frame "Module" {
            n185 = call-poly <vilib>:"Read Key.vi"("section"=w397, "key"="Path", "refnum"=w403) -> ("error out"=w401:errorcluster, "value"=w394:string, "refnum out"=w402:T1)  [unwired: 5 in, 1 out]
            n186 = call "GetSectionData.vi"("SectionName"=w397, "error in"=w401, "ConfigRef"=w402) -> ("error out"=w399:errorcluster, "Data"=w392:string[][])  [unwired: 6 in, 1 out]
            n187 = Build Array (concatenate)(w390, w392) -> (w391:string[][])
            n188 = call "FixMacPath.vi"("Input Path String"=w394) -> ("Output Path"=w393:path)  [unwired: 4 in]
            n189 = To Variant(anything=w391) -> (Variant=w398:variant)
            n190 = case shown="\"Development System\"" w396 {
              tunnel: [w405 w408] -> w395
              tunnel: w393 -> [w404 w409]
              frame "Run Time System", Default {
                n191 = Current VI's Path() -> (path=w407:path)
                n192 = Strip Path(path=w407) -> (stripped path=w406:path)  [unwired: 1 out]
                n193 = Build Path(base path=w406, name or relative path=w404) -> (appended path=w405:path)
              }
              frame "Development System" {
                n194 = call <userlib>:"Current VIs Parent Directory__ogtk.vi"("Relative path (.)"=w409) -> ("Parent Directory (+ Relative)"=w408:path)  [unwired: 4 in]
              }
            }
          }
          frame "Plot" {
            # "Custom Plot"
            n195 = Index Array(array=w417, index (dim 0)=w413) -> (element=w411:string[][])  [unwired: 2 in]
            n196 = Build Array (concatenate)(w412, w411) -> (w410:string[][])
            n197 = To Variant(anything=w410) -> (Variant=w416:variant)
            n198 = case shown="\"Run Time System\", Default" w414 {
              tunnel: [w420 path "Support/SubPanel/Plot/Plot.vi"] -> w415
              frame "Run Time System", Default {
                n199 = call "FixMacPath.vi"("Input Path String"="..\\Support\\SubPanel\\Plot\\Plot.vi" ("value")) -> ("Output Path"=w418:path)  [unwired: 4 in]
                n200 = Current VI's Path() -> (path=w421:path)
                n201 = Build Path(base path=w421, name or relative path=w418) -> (appended path=w420:path)
              }
              frame "Development System" {
              }
            }
          }
          frame "Binary Plot" {
            # "Custom Plot"
            n202 = Index Array(array=w430, index (dim 0)=w426) -> (element=w425:string[][])  [unwired: 2 in]
            n203 = Build Array (concatenate)(w423, w425) -> (w424:string[][])
            n204 = To Variant(anything=w424) -> (Variant=w429:variant)
            n205 = case shown="\"Run Time System\", Default" w427 {
              tunnel: [w433 path "Support/SubPanel/BinaryPlot/BinaryPlot.vi"] -> w428
              frame "Run Time System", Default {
                n206 = call "FixMacPath.vi"("Input Path String"="..\\Support\\SubPanel\\BinaryPlot\\BinaryPlot.vi" ("value")) -> ("Output Path"=w431:path)  [unwired: 4 in]
                n207 = Current VI's Path() -> (path=w434:path)
                n208 = Build Path(base path=w434, name or relative path=w431) -> (appended path=w433:path)
              }
              frame "Development System" {
              }
            }
          }
        }
        n209 = Open VI Reference(vi path=w361, error in (no error)=w366) -> (vi reference=w380:refnum<vi>, error out=w364:errorcluster)  [unwired: 4 in]
        n210 = Path To String(path=w361) -> (string=w360:string)
        n211 = Bundle By Name(cluster=w364, "source"=w360) -> (w363:errorcluster)
        n212 = invoke class="VI" method="Run VI"(reference=w380, error in=w363, "Wait until done"=FALSE ("Wait Until Done")) -> (reference out=w368:refnum<vi>, error out=w375:errorcluster)  [unwired: 2 in, 3 out]
        n213 = call "NextState.vi"("Error In"=w375, "Data"=w372, "State"="Initialize", "Queue In"=w367) -> ("Error Out"=w370:errorcluster)  [unwired: 6 in, 1 out]
        n214 = Merge Errors(w369, w370) -> (w371:errorcluster)
        n215 = invoke on="Sub Panel" class="SubPanel" method="Insert VI"(error in=w371, "VI Ref"=w368) -> (error out=w378:errorcluster)  [unwired: 2 in, 3 out]
        n216 = property on="Parameter Type" class="Ring (strict)"("DisabledEnum"=w347) -> ()  [unwired: 2 in, 2 out]
        n217 = call "NextState.vi"("State"="Default Timeout", "Queue In"=w355) -> ()  [unwired: 8 in, 2 out]
        n218 = Bundle By Name(cluster=w382, "Error"=w378, "SubPanel"=w368) -> (w381:T2)
        n219 = property on="Upload" class="Bool"("DisabledEnum"=w347) -> ()  [unwired: 2 in, 2 out]
      }
      frame "--- Communication ---" {
      }
      frame "Update Comm Controls" {
        w439 = "Configuration" ("section")
        # "In addition to comm controls,\nupdate commands/telemetry"
        n220 = Unbundle By Name(w438) -> ("ConfigRef"=w442:T1)
        n221 = call <vilib>:"Get Key Names.vi"("section"=w439, "refnum"=w442) -> ("key names"=w441:string[], "refnum out"=w440:T1)  [unwired: 6 in, 2 out]
        n222 = for {
          tunnel: w441 -> [w446] mode=indexing
          tunnel: w440 -> [w448]
          tunnel: w439 -> [w447]
          shift-right: [w443] -> w437
          shift-left: w438 -> [w444]
          n223 = call-poly <vilib>:"Read Key.vi"("section"=w447, "key"=w446, "refnum"=w448) -> ("value"=w445:string)  [unwired: 5 in, 3 out]
          n224 = case shown="\"StartUpDelay\"" w446 {
            tunnel: w445 -> [_ w451 w453 w456 w457 w460 w463 w469]
            tunnel: w444 -> [w449 w450 w452 w455 w458 w461 w465 w468]
            tunnel: [w449 w450 w452 w455 w459 w462 w464 w467] -> w443
            frame Default {
            }
            frame "COMport" {
              n225 = local write "*Com Port"(w451) -> ()
            }
            frame "Timeout" {
              n226 = Fract/Exp String To Number(string=w453) -> (number=w454:dbl)  [unwired: 3 in, 1 out]
              n227 = local write "*Timeout (sec)"(w454) -> ()
            }
            frame "Baud" {
              n228 = local write "*Baud Rate"(w456) -> ()
            }
            frame "Version" {
              n229 = Bundle By Name(cluster=w458, "Version"=w457) -> (w459:T2)
            }
            frame "StopTelem" {
              n230 = Bundle By Name(cluster=w461, "StopTelem"=w460) -> (w462:T2)
            }
            frame "SW" {
              n231 = Bundle By Name(cluster=w465, "SW"=w463) -> (w464:T2)
            }
            frame "StartUpDelay" {
              n232 = Fract/Exp String To Number(string=w469) -> (number=w466:dbl)  [unwired: 3 in, 1 out]
              n233 = local write "*BootDelay"(w466) -> ()
              n234 = Bundle By Name(cluster=w468, "StartDelay"=w466) -> (w467:T2)
            }
          }
        }
      }
      frame "Save Comm Controls" {
        n235 = Unbundle By Name(w470) -> ("ConfigRef"=w472:T1)
        n236 = for {
          tunnel: string[] ["COMport", "Timeout", "Baud", "StartUpDelay"] -> [w475] mode=indexing
          tunnel: w472 -> [w477]
          tunnel: "Configuration" ("section") -> [w476]
          n237 = case shown="\"StartUpDelay\"" w475 {
            tunnel: [_ w478 w479 w481 w482] -> w474
            frame Default {
            }
            frame "COMport" {
              n238 = local read "*Com Port"() -> (w478:refnum<visa-resource-name>)
            }
            frame "Timeout" {
              n239 = local read "*Timeout (sec)"() -> (w480:dbl)
              n240 = Number To Fractional String(number=w480) -> (F-format string=w479:string)  [unwired: 3 in]
            }
            frame "Baud" {
              n241 = local read "*Baud Rate"() -> (w481:string)
            }
            frame "StartUpDelay" {
              n242 = local read "*BootDelay"() -> (w483:dbl)
              n243 = Number To Fractional String(number=w483) -> (F-format string=w482:string)  [unwired: 3 in]
            }
          }
          n244 = call-poly <vilib>:"Write Key.vi"("section"=w476, "value"=w474, "key"=w475, "refnum"=w477) -> ()  [unwired: 5 in, 3 out]
        }
      }
      frame "Lock Comm Controls" {
        w484 = T3."Disabled and Grayed Out" ("Disabled")
        n245 = property on="*Com Port" class="VISAName"("DisabledEnum"=w484) -> ()  [unwired: 2 in, 2 out]
        n246 = property on="*Baud Rate" class="CmbBox"("DisabledEnum"=w484) -> ()  [unwired: 2 in, 2 out]
        n247 = property on="*Timeout (sec)" class="DigNum (strict)"("DisabledEnum"=w484) -> ()  [unwired: 2 in, 2 out]
        n248 = property on="*BootDelay" class="DigNum (strict)"("DisabledEnum"=w484) -> ()  [unwired: 2 in, 2 out]
      }
      frame "Unlock Comm Controls" {
        w486 = T3."Enabled" ("Disabled")
        n249 = property on="*Com Port" class="VISAName"("DisabledEnum"=w486) -> ()  [unwired: 2 in, 2 out]
        n250 = property on="*Baud Rate" class="CmbBox"("DisabledEnum"=w486) -> ()  [unwired: 2 in, 2 out]
        n251 = property on="*Timeout (sec)" class="DigNum (strict)"("DisabledEnum"=w486) -> ()  [unwired: 2 in, 2 out]
        n252 = property on="*BootDelay" class="DigNum (strict)"("DisabledEnum"=w486) -> ()  [unwired: 2 in, 2 out]
      }
      frame "Update Termination Character" {
        n253 = Unbundle By Name(w491) -> ("COM Port"=w490:refnum<visa-resource-name>)
        n254 = Variant To Data(Variant=w492, type=u8 10 ("termination char\n(0xA = '\\n' = LF)")) -> (data=w488:u8)  [unwired: 1 in, 1 out]
        n255 = property class="Instr"(reference=w490, "TermChar"=w488) -> ()  [unwired: 1 in, 2 out]
      }
      frame "Remote Open Port" {
        n256 = Variant To Data(Variant=w496, type="") -> (data=w494:string)  [unwired: 1 in, 1 out]
        n257 = case shown="Default" w494 {
          selector: w494 -> [_ w500]
          tunnel: w493 -> [_ w498]
          frame "" {
          }
          frame Default {
            n258 = local write "*Com Port"(w500) -> ()
            n259 = call "NextState.vi"("State"="Open Port", "Queue In"=w498) -> ()  [unwired: 8 in, 2 out]
          }
        }
      }
      frame "Open Port" {
        n260 = Unbundle By Name(w503) -> ("ConnType"=w502:string)
        n261 = Match Pattern(string="*Com Port", regular expression="TCPIP") -> (offset past match=w504:i32)  [unwired: 1 in, 3 out]
        n262 = case shown="-1" w504 {
          tunnel: [w517 w523] -> w515
          tunnel: [_ w522] -> w512
          tunnel: "*Com Port" -> [w517 w524]
          tunnel: "*BootDelay" -> [_ w520]
          frame Default {
            # "TCP Connection"
          }
          frame -1 {
            w533 = u16 0 items=["None", "XON/XOFF", "RTS/CTS", "XON/XOFF & RTS/CTS", "DTR/DSR", "XON/XOFF & DTR/DSR"] ("flow control (0:none)")
            n263 = Decimal String To Number(string="*Baud Rate", default (0L)=u32 0 ("default (0 I32)")) -> (number=w528:u32)  [unwired: 1 in, 1 out]
            n264 = call-poly "VISA Configure Serial Port"("VISA resource name"=w524, "timeout (10sec)"=u32 1000, "termination char\n(0xA = '\\n' = LF)"=u8 10 ("termination char\n(0xA = '\\n' = LF)"), "Enable Termination\nChar (T)"=TRUE ("Enable Termination\nChar (T)"), "baud rate (9600)"=w528, "flow control (0:none)"=w533) -> ("VISA resource name out"=w518:refnum<visa-resource-name>, "error out"=w521:errorcluster)  [unwired: 3 in, 5 out]
            n265 = call "Time Delay9"("error in (no error)"=w521, "Delay Time (s)"=w520) -> ("error out"=w519:errorcluster)  [unwired: 9 in]
            n266 = VISA Set I/O Buffer Size(VISA resource name=w518, size (4096)=u32 64000, error in (no error)=w519) -> (VISA resource name out=w531:refnum<visa-resource-name>, error out=w532:errorcluster)  [unwired: 1 out]
            n267 = property class="Instr"(reference=w531, error in=w532, "Timeout"=u32 1000 ("General Settings:Timeout Value")) -> (reference out=w523:refnum<visa-resource-name>, error out=w522:errorcluster)
          }
        }
        n268 = local write "Status"("Please Wait, Connecting to the AeroQuad..." ("Status")) -> ()
        n269 = call "NextState.vi"("State"="Lock User Controls", "Queue In"=w508) -> ("Queue Out"=w509:refnum<queue>)  [unwired: 8 in, 1 out]
        n270 = call "NextState.vi"("Error In"=w512, "State"=w502, "Queue In"=w509) -> ()  [unwired: 7 in, 2 out]
        n271 = property on="Open Port" class="Bool"(error in=w512, "DisabledEnum"=T3."Disabled and Grayed Out" ("Disabled")) -> (error out=w507:errorcluster)  [unwired: 1 in, 1 out]
        n272 = Bundle By Name(cluster=w503, "COM Port"=w515, "Error"=w507) -> (w516:T2)
        n273 = local write "Sensors"(string[][] [] ("Sensors")) -> ()
      }
      frame "Check Connection" {
        n274 = Unbundle By Name(w545) -> ("Logger"=w536:bool, "DebugLogger"=w537:refnum<queue>, "COM Port"=w541:refnum<visa-resource-name>, "SW"=w548:string, "Compatibility"=w538:dbl)
        n275 = call "NextState.vi"("State"="Connect", "Queue In"=w546) -> ()  [unwired: 8 in, 2 out]
        n276 = while {
          tunnel: w541 -> [w565]
          tunnel: w548 -> [w551]
          shift-right: [w563] -> w539
          shift-left: errorcluster {"status"=FALSE, "code"=0, "source"=""} ("error out") -> [w564]
          tunnel: "*Timeout (sec)" -> [w558]
          shift-right: [w555] -> _
          shift-left: TRUE -> [w556]
          tunnel: [w554] -> _
          tunnel: w538 -> [w553]
          tunnel: w537 -> [w552]
          tunnel: w536 -> [w549]
          i -> [w554]
          stop <- w555 stop-if-true
          n277 = VISA Write(VISA resource name=w565, write buffer=w551, error in (no error)=w564) -> (VISA resource name out=w559:refnum<visa-resource-name>, error out=w566:errorcluster)  [unwired: 1 out]
          n278 = call "Time Delay4"("error in (no error)"=w566) -> ("error out"=w560:errorcluster)  [unwired: 1 in, 9 out]
          n279 = VISA Read(VISA resource name=w559, byte count=u32 1024, error in (no error)=w560) -> (VISA resource name out=w561:refnum<visa-resource-name>, read buffer=w550:string, error out=w562:errorcluster)  [unwired: 1 out]
          n280 = case shown="True" w549 {
            tunnel: w552 -> [_ w571]
            tunnel: w551 -> [_ w570]
            tunnel: w550 -> [_ w567]
            frame False {
            }
            frame True {
              n281 = call "NextState.vi"("Data"=w570, "State"="Write", "Queue In"=w571) -> ("Queue Out"=w568:refnum<queue>)  [unwired: 7 in, 1 out]